vi "UHR-Fleezers Control (host) - 10.2.vi"() -> ()   [LabVIEW 2009] (continued)
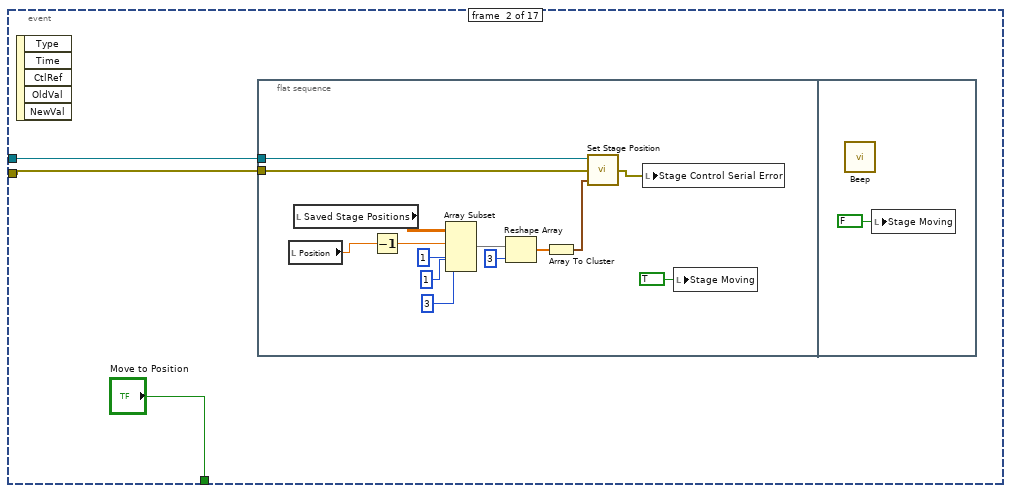
[diagram p2: hidden frame]
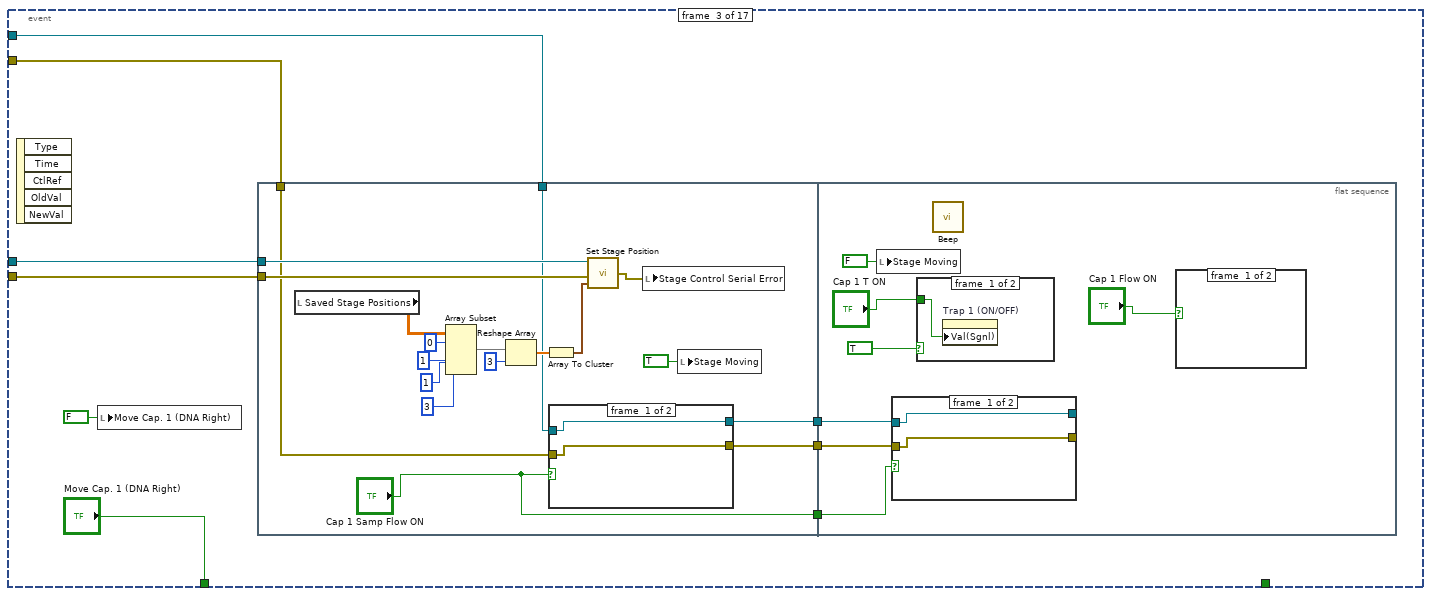
[diagram p3: hidden frame]
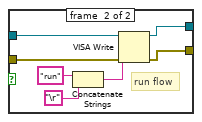
[diagram p4: hidden frame]
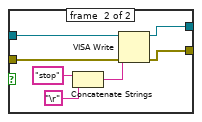
[diagram p5: hidden frame]
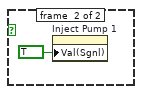
[diagram p6: hidden frame]
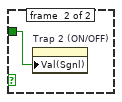
[diagram p7: hidden frame]
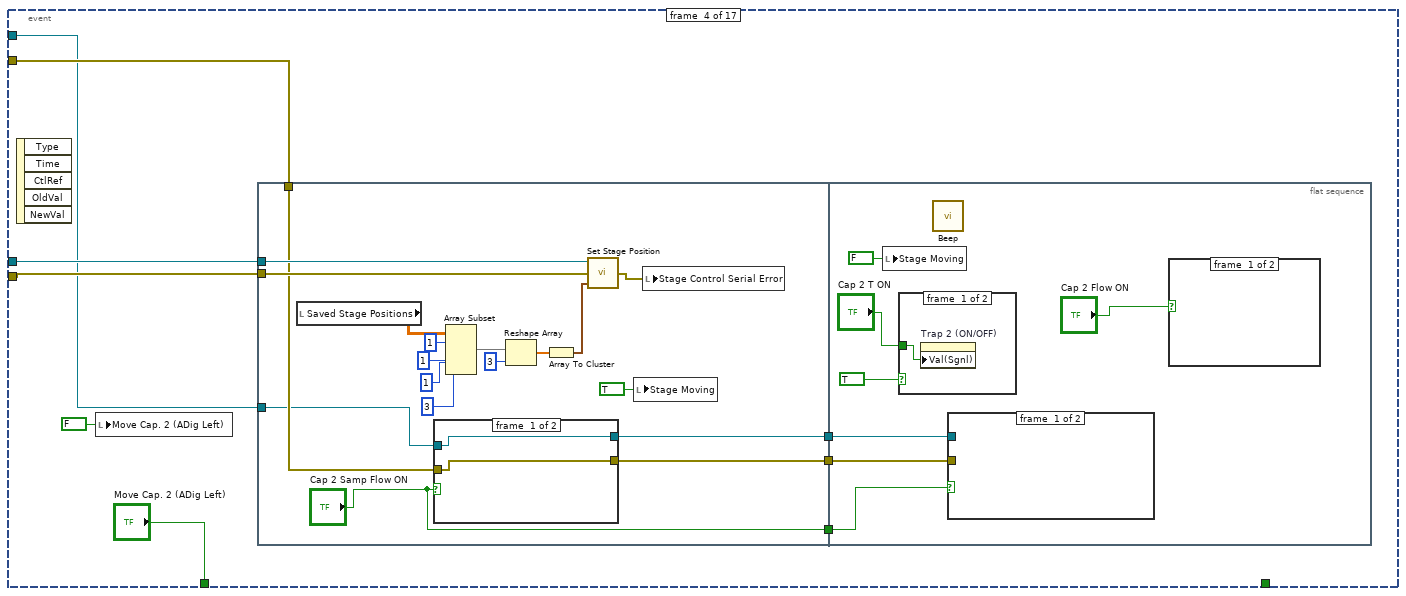
[diagram p8: hidden frame]
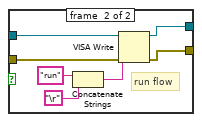
[diagram p9: hidden frame]
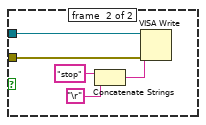
[diagram p10: hidden frame]
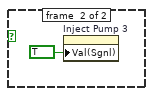
[diagram p11: hidden frame]
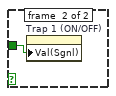
[diagram p12: hidden frame]
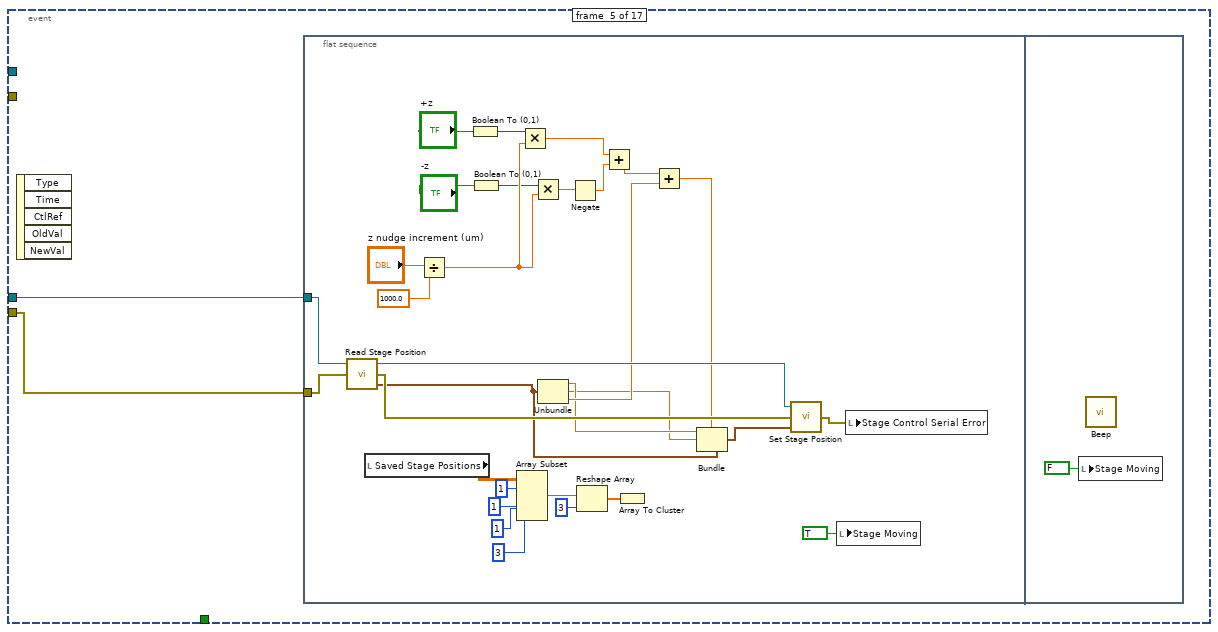
[diagram p13: hidden frame]
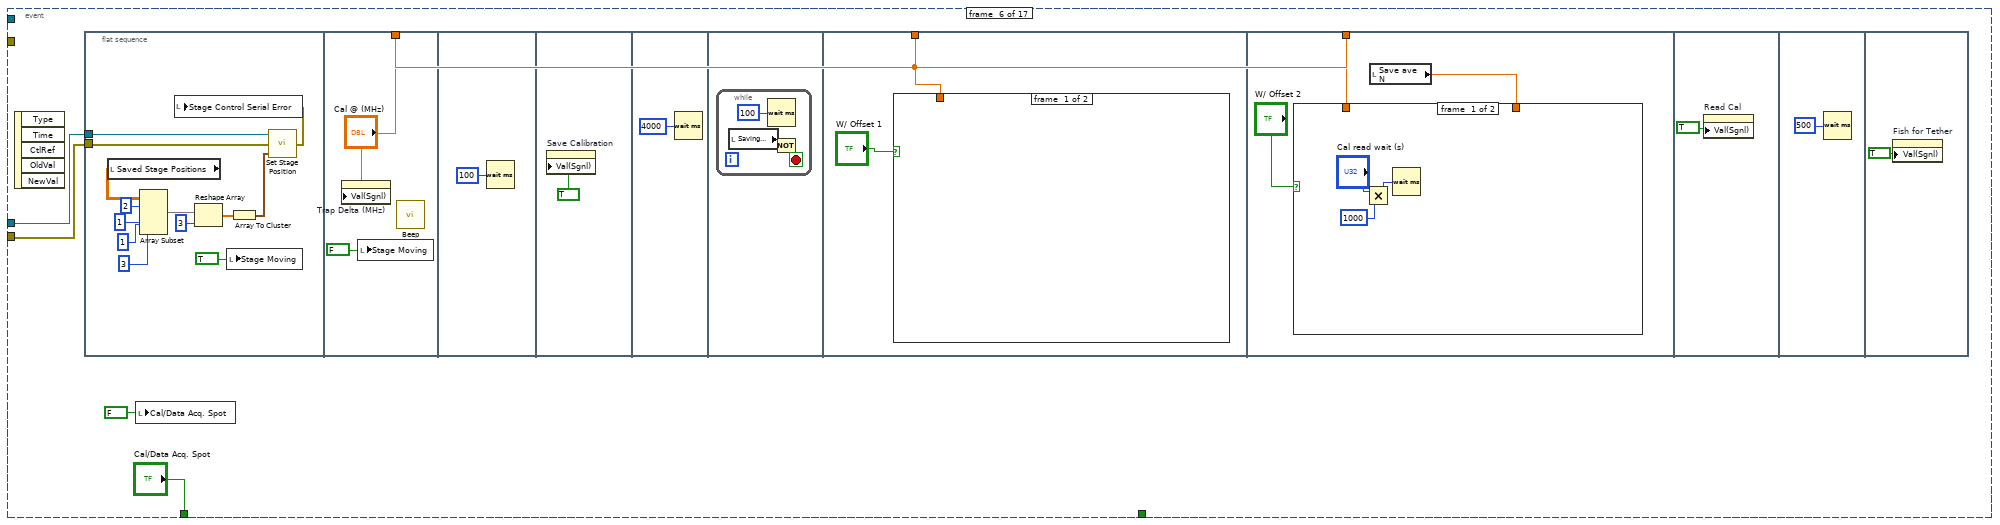
[diagram p14: hidden frame]
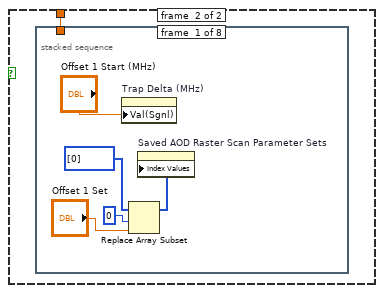
[diagram p15: hidden frame]
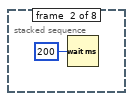
[diagram p16: hidden frame]
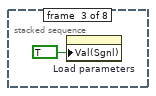
[diagram p17: hidden frame]
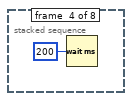
[diagram p18: hidden frame]
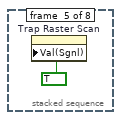
[diagram p19: hidden frame]
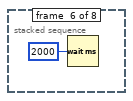
[diagram p20: hidden frame]
              frame #0 {
              }
              frame #1 {
                n2014 = call "IMAQ AVI Close"("Avi Refnum"=w8057) -> ()  [unwired: 1 in, 10 out]
              }
            }
            n2015 = call "IMAQ AVI Create"("Frames Per Second"=u32 30, "AVI Path"=w8046) -> ("Avi Refnum"=w8054:T48)  [unwired: 5 in, 4 out]
            n2016 = local write "Video Index"(w8056) -> ()
          }
        }
        n2017 = Equal To 0?(x=w8037) -> (x = 0?=w8036:bool)
        n2018 = Select(t=w8027, s=w8028, f=w8025) -> (s? t:f=w8026:T48)
        n2019 = case shown="True" w8036 {
          tunnel: w8035 -> [w8058 w8083]
          tunnel: w8034 -> [_ w8082]
          tunnel: [w8058 w8079] -> w8032
          tunnel: w8031 -> [_ w8063]
          tunnel: w8020 -> [_ w8067]
          tunnel: w8026 -> [_ w8065]
          tunnel: w8018 -> [_ w8060]
          tunnel: w8017 -> [_ w8059]
          frame #0 {
          }
          frame #1 {
            w8073 = u32 0 ("X-offset IN")
            n2020 = call "DMR_GetImageRequestBufferData.vi"("driver handle IN"=w8083, "request number IN"=w8082) -> ("width OUT"=w8072:i32, "height OUT"=w8071:i32, "driver handle OUT"=w8078:i32, "request number OUT"=w8077:i32, "bytes per pixel OUT"=w8074:i32)  [unwired: 13 out]
            n2021 = call "DMR_GetImageRequestBufferImageData.vi"("driver handle IN"=w8078, "request number IN"=w8077, "bytes per pixel IN"=w8074, "X-offset IN"=w8073, "Y-offset IN"=w8073, "height IN"=w8071, "width IN"=w8072) -> ("driver handle OUT"=w8076:u32, "request number OUT"=w8075:u32, "image OUT"=w8068:u32[][])  [unwired: 10 out]
            n2022 = call "DMR_ImageRequestUnlock.vi"("request number IN"=w8075, "driver handle IN"=w8076) -> ("driver handle OUT"=w8081:i32)  [unwired: 1 in, 2 out]
            n2023 = case shown="True" "Averaging" {
              tunnel: w8068 -> [w8119 w8124]
              tunnel: [w8119 w8123] -> w8064
              tunnel: w8067 -> [_ w8121]
              frame #0 {
              }
              frame #1 {
                (unwired) 1
                w8129 = 1
                n2024 = feedback #32(w8121) -> (w8120:u32[][])
                n2025 = Add(x=w8124, y=w8120) -> (x+y=w8125:u32[][])
                n2026 = Select(t=w8121, s="Reset Averaging", f=w8125) -> (s? t:f=w8127:u32[][])
                n2027 = feedback #33(w8129) -> (w8122:i32)
                n2028 = Divide(x=w8125, y=w8122) -> (x/y=w8126:dbl[][])
                n2029 = Increment(x=w8122) -> (x+1=w8130:i32)
                n2030 = To Unsigned Long Integer(number=w8126) -> (unsigned 32bit integer=w8123:u32[][])
                n2031 = Select(t=w8129, s="Reset Averaging", f=w8130) -> (s? t:f=w8128:i32)
              }
            }
            n2032 = call "DMR_ImageRequestSingle.vi"("request control IN"=0, "driver handle IN"=w8081) -> ("driver handle OUT"=w8079:i32)  [unwired: 3 out]
            n2033 = disable-structure shown="Disabled" {
              disable-tunnel: w8064 -> [w8096 _]
              disable-tunnel: w8060 -> [w8095 _]
              frame #0 {
                n2034 = To Double Precision Float(number=w8096) -> (double precision float=w8094:dbl[][])
                n2035 = In Range and Coerce(upper limit="Intensity Upper", x=w8094, lower limit="Intensity Lower") -> (coerced(x)=w8093:dbl[][])  [unwired: 1 out]
                n2036 = Subtract(x="Intensity Upper", y="Intensity Lower") -> (x-y=w8090:dbl)
                n2037 = Subtract(x=w8093, y="Intensity Lower") -> (x-y=w8091:dbl[][])
                n2038 = Divide(x=w8091, y=w8090) -> (x/y=w8092:dbl[][])
                n2039 = Multiply(x=255.0, y=w8092) -> (x*y=w8088:dbl[][])
                n2040 = To Unsigned Byte Integer(number=w8088) -> (unsigned 8bit integer=w8097:u8[][])
                n2041 = call "IMAQ ArrayToImage"("Image Pixels (U8)"=w8097, "Image"=w8095) -> ("Image Out"=w8084:T2)  [unwired: 4 in, 5 out]
                n2042 = First Call?() -> (First Call?: T/F=w8085:bool)
                n2043 = case shown="True" w8085 {
                  tunnel: w8084 -> [w8098 w8109]
                  frame #0 {
                    n2044 = flat-sequence {
                      tunnel: w8098 -> [w8104]
                      frame #0 {
                        w8101 = FALSE ("Get/Set Status? (Set)")
                        w8100 = 0 ("Window Number (0...15)")
                        n2045 = call "IMAQ WindSize"("Get/Set Status? (Set)"=w8101, "Window Number"=w8100) -> ("Width & Height out"=→"Window Size":cluster{"Width":i32, "Height":i32})  [unwired: 4 in, 2 out]
                        n2046 = call "IMAQ WindMove"("Window Number (0...15)"=w8100, "Get/Set Status? (Set)"=w8101) -> ("Coordinates (screen)"=→"Window Position":cluster{"X Position":i32, "Y Position":i32})  [unwired: 3 in, 1 out]
                        n2047 = call "IMAQ WindDraw"("Resize to Image Size? (Y)"=FALSE, "Window Number (0...15)"=w8100, "Image"=w8104) -> ()  [unwired: 7 in, 2 out]
                      }
                      frame #1 {
                        n2048 = call "IMAQ WindZoom 2"("Center Point"="Center Point", "Zoom to Fit? (False)"=FALSE, "Zoom Factor"="Zoom Factor") -> ()  [unwired: 5 in, 4 out]
                      }
                    }
                  }
                  frame #1 {
                    n2049 = flat-sequence {
                      tunnel: w8109 -> [w8112]
                      tunnel: [w8110] -> w8108
                      tunnel: w8108 -> [w8114]
                      frame #0 {
                        w8111 = TRUE ("Resize to Image Size? (Y)")
                        w8110 = 0 ("Window Number (0...15)")
                        n2050 = call "IMAQ WindNonTearing"("Window Number"=w8110, "NonTearing? (True)"=w8111) -> ()  [unwired: 8 in, 2 out]
                        n2051 = call "IMAQ WindDraw"("Resize to Image Size? (Y)"=w8111, "Window Number (0...15)"=w8110, "Image"=w8112) -> ()  [unwired: 7 in, 2 out]
                      }
                      frame #1 {
                        n2052 = call "IMAQ WindSize"("Scrollbars? (N)"=FALSE, "Width & Height"="Initial Window Size", "Window Number"=w8114) -> ()  [unwired: 3 in, 3 out]
                        n2053 = call "IMAQ WindMove"("Window Number (0...15)"=w8114, "Coordinates (screen)"="Initial Window Position") -> ()  [unwired: 3 in, 2 out]
                      }
                    }
                  }
                }
              }
              frame #1 {
              }
            }
            n2054 = To Unsigned Byte Integer(number=w8064) -> (unsigned 8bit integer=w8062:u8[][])
            n2055 = call "IMAQ ArrayToImage"("Image Pixels (U8)"=w8062, "Image"=w8063) -> ("Image Out"=w8061:T2)  [unwired: 4 in, 5 out]
            "Primary Video Display" <- w8061
            n2056 = case shown="True" "Save Video" {
              tunnel: w8065 -> [_ w8118]
              tunnel: w8061 -> [_ w8117]
              frame #0 {
              }
              frame #1 {
                n2057 = call "IMAQ AVI Write Frame"("Image"=w8117, "Avi Refnum"=w8118) -> ()  [unwired: 2 in, 8 out]
              }
            }
            n2058 = case shown="True" "Save Image" {
              tunnel: w8062 -> [_ w8133]
              tunnel: w8059 -> [_ w8132]
              frame #0 {
              }
              frame #1 {
                n2059 = call <vilib>:"Flatten Pixmap.vi"("colors"=w8132, "8-bit pixmap"=w8133) -> ("image data"=w8139:T49)  [unwired: 4 in, 5 out]
                n2060 = call "Create new save file.vi"("Insert"="video_frame_" ("string"), "Ext"=".bmp" ("string"), "Index In"="Image Index") -> ("Path Out"=w8135:path, "Index Out"=w8140:dbl)
                n2061 = Increment(x=w8140) -> (x+1=w8134:dbl)
                n2062 = local write "Image Index"(w8134) -> ()
                n2063 = call <vilib>:"Write BMP File.vi"("image data"=w8139, "path to BMP file"=w8135) -> ()  [unwired: 1 in, 9 out]
              }
            }
          }
        }
        n2064 = node-c288(w8021) -> ()  [unwired: 1 out]
      }
      n2065 = node-c288(w8005) -> ()  [unwired: 1 out]
      n2066 = call "DMR_CloseDevice.vi"("driver handle IN"=w8010) -> ()  [unwired: 1 in, 4 out]
    }
    frame #4 {
      n2067 = call "DMR_Close.vi"() -> ()  [unwired: 1 out]
    }
  }
  n2068 = timed-loop "Oscillate AOD (debugging)" {
    tunnel: w8 -> [w8146]
    tunnel: [w8145] -> w53
    timing: w48 -> [_]
    timing-out: [_] -> w47
    stop <- w8145 stop-if-true
    n2069 = node-c288() -> ()  [unwired: 2 out]
    n2070 = event shown="[0] \"Oscillate Set 1\", \"Fish for Tether\": Value Change" {
      selector: _ -> [_ _ _]
      dyn-events: _ -> [_ _ _]
      timeout: _ -> [_ _ _]
      tunnel: w8146 -> [w8153 _ _]
      tunnel: [FALSE ("Stop All") _ w8421] -> w8145
      event #0 {
        n2071 = event-data() -> ()  [unwired: 6 out]
        n2072 = local read "Oscillate Set 1"() -> (w8152:bool)
        n2073 = Or(x=w8152, y="Fish for Tether") -> (x .or. y?=w8150:bool)
        n2074 = case shown="True" w8150 {
          tunnel: w8153 -> [_ w8155]
          tunnel: "Fish for Tether" -> [_ w8154]
          frame #0 {
          }
          frame #1 {
            n2075 = case shown="True" w8154 {
              frame #0 {
              }
              frame #1 {
                n2076 = local write "Scan axis 2"(TRUE) -> ()
                n2077 = local write "Tether"(FALSE ("Tether")) -> ()
              }
            }
            n2078 = node-c288() -> (w8157:T23)  [unwired: 4 out]
            n2079 = timed-loop "Oscillate AOD" {
              timing: w8157 -> [_]
              timing-out: [_] -> w8156
              tunnel: w8155 -> [w8167]
              tunnel: w8154 -> [w8166]
              i -> [w8169]
              stop <- w8165 stop-if-true
              n2080 = node-c288() -> (w8168:i64)  [unwired: 1 out]
              n2081 = flat-sequence {
                tunnel: w8169 -> [w8196]
                tunnel: w8168 -> [w8195]
                tunnel: w8167 -> [w8174]
                tunnel: w8166 -> [w8177]
                tunnel: [w8177] -> w8164
                tunnel: [w8176] -> w8163
                tunnel: [w8173] -> w8162
                tunnel: [w8170] -> w8160
                tunnel: w8164 -> [w8232]
                tunnel: w8163 -> [w8230]
                tunnel: w8162 -> [w8229]
                tunnel: [w8228] -> w8161
                tunnel: w8160 -> [w8227]
                tunnel: [w8295] -> w8165
                tunnel: w8161 -> [w8294]
                frame #0 {
                  n2082 = Divide(x=w8195, y=i64 1000) -> (x/y=w8190:dbl)
                  n2083 = Multiply(x=w8190, y=w8196) -> (x*y=w8192:dbl)
                  n2084 = local read "BD 1 Frequency 2 (MHz)"() -> (w8175:dbl)
                  n2085 = Multiply(x="Osc. freq. (Hz)", y=6.283185307179586) -> (x*y=w8193:dbl)
                  n2086 = Multiply(x=w8193, y=w8192) -> (x*y=w8172:dbl)
                  n2087 = local read "BD 1 Frequency 1 (MHz)"() -> (w8180:dbl)
                  n2088 = case shown="True" w8177 {
                    tunnel: w8172 -> [w8202 w8207]
                    tunnel: w8180 -> [_ w8218]
                    tunnel: w8175 -> [_ w8219]
                    tunnel: [w8199 w8213] -> w8178
                    tunnel: [FALSE w8210] -> w8173
                    tunnel: [0.0 w8203] -> w8170
                    frame #0 {
                      n2089 = Sine(x=w8202) -> (sin(x)=w8200:dbl)
                      n2090 = Multiply(x=w8200, y="Osc. amp. (MHz)") -> (x*y=w8199:dbl)
                    }
                    frame #1 {
                      n2091 = Cosine(x=w8207) -> (cos(x)=w8222:dbl)
                      n2092 = Subtract(x=w8219, y=w8218) -> (x-y=w8217:dbl)
                      n2093 = Decrement(x=w8222) -> (x-1=w8221:dbl)
                      n2094 = Subtract(x=w8217, y="Closest Delta (MHz)") -> (x-y=w8214:dbl)
                      n2095 = Divide(x=w8221, y=-2.0) -> (x/y=w8215:dbl)
                      n2096 = Multiply(x=w8215, y=w8214) -> (x*y=w8213:dbl)
                      n2097 = local read "Vec Mean of T1 T2"() -> (w8209:dbl[])
                      n2098 = Greater?(x=w8209, y="Stop F (pN)") -> (0:w8211:bool[])
                      n2099 = Or Array Elements(Boolean array=w8211) -> (logical OR=w8210:bool)
                      n2100 = Divide(x=w8207, y=6.283185307179586) -> (x/y=w8206:dbl)
                      n2101 = Round Toward +Infinity(x=w8206) -> (ceil(x): smallest int >= x=w8203:dbl)
                      "Attempts" <- w8203
                      n2102 = Greater?(x=w8203, y="Attempt Limit") -> (0:w8205:bool)
                      n2103 = case shown="True" w8205 {
                        frame #0 {
                        }
                        frame #1 {
                          n2104 = call <vilib>:"Beep.vi"() -> ()  [unwired: 3 in, 9 out]
                          n2105 = local write "Fish for Tether"(FALSE ("Fish for Tether")) -> ()
                          n2106 = local read "Messages"() -> (w8224:string)
                          n2107 = call "Update messages.vi"("Message to add"="Tether fishing timeout." ("Messages"), "Old message string"=w8224) -> ("New message string"=→"Messages":string)
                        }
                      }
                    }
                  }
                  n2108 = local read "BD 2 Frequency 1 (MHz)"() -> (w8179:dbl)
                  n2109 = Select(t=w8180, s="Scan axis 2", f=w8179) -> (s? t:f=w8183:dbl)
                  n2110 = Add(x=w8178, y=w8183) -> (x+y=w8176:dbl)
                  n2111 = Select(t=w8176, s="Scan axis 2", f=w8180) -> (s? t:f=w8186:dbl)
                  n2112 = Select(t=w8179, s="Scan axis 2", f=w8176) -> (s? t:f=w8185:dbl)
                  n2113 = local read "Y RF Frequency Limits (MHz)"() -> (w8181:T16)
                  n2114 = local read "X RF Frequency Limits (MHz)"() -> (w8182:T16)
                  n2115 = local read "BD 1 Frequency 3 (MHz)"() -> (w8189:dbl)
                  n2116 = local read "BD 2 Frequency 2 (MHz)"() -> (w8188:dbl)
                  n2117 = local read "BD 2 Frequency 3 (MHz)"() -> (w8187:dbl)
                  n2118 = call "set RF board frequency - interlace.vi"("Board 2 Frequency Limits"=w8181, "Board 1 Frequency Limits"=w8182, "FPGA VI Reference In"=w8174, "Board 2 Frequency 3 (MHz)"=w8187, "Board 1 Frequency 3 (MHz)"=w8189, "Board 2 Frequency 2 (MHz)"=w8188, "Board 2 Frequency 1 (MHz)"=w8185, "Board 1 Frequency 2 (MHz)"=w8175, "Board 1 Frequency 1  (MHz)"=w8186) -> ()  [unwired: 1 in, 2 out]
                }
                frame #1 {
                  n2119 = And(x=w8232, y=w8229) -> (x .and. y?=w8231:bool)
                  n2120 = case "Only if were fishing and now formed tether" shown="True" w8231 {
                    tunnel: w8230 -> [w8234 w8247]
                    tunnel: [w8233 w8246] -> w8228
                    tunnel: w8227 -> [_ w8242]
                    frame #0 {
                      n2121 = local read "Fish for Tether"() -> (w8233:bool)
                      n2122 = case shown="False" w8233 {
                        tunnel: w8234 -> [w8235 _]
                        frame #0 {
                          n2123 = property on="BD 1 Frequency 1 (MHz)" class="DigNum (strict)"("Val(Sgnl)"=w8235) -> ()  [unwired: 2 in, 2 out]
                        }
                        frame #1 {
                        }
                      }
                    }
                    frame #1 {
                      w8246 = FALSE ("Fish for Tether")
                      n2124 = call <vilib>:"Beep.vi"() -> ()  [unwired: 3 in, 9 out]
                      n2125 = Number To Decimal String(number=w8242, width (-)=i16 1) -> (decimal integer string=w8240:string)
                      n2126 = case shown="\"2\", \"3\", \"4\", \"5\", \"6\"" "Then..." {
                        selector: "Then..." -> [_ w8250]
                        tunnel: w8247 -> [w8249 _]
                        frame #0 {
                          n2127 = property on="BD 1 Frequency 1 (MHz)" class="DigNum (strict)"("Val(Sgnl)"=w8249) -> ()  [unwired: 2 in, 2 out]
                        }
                        frame #1 {
                          n2128 = flat-sequence {
                            tunnel: w8250 -> [w8252]
                            frame #0 {
                              n2129 = property on="Trap Delta (MHz)" class="DigNum (strict)"("Val(Sgnl)"="Move to Delta 1 (MHz)") -> ()  [unwired: 2 in, 2 out]
                            }
                            frame #1 {
                              n2130 = case shown="\"5\", \"6\"" w8252 {
                                selector: w8252 -> [w8255 w8265 _]
                                frame #0 {
                                n2131 = flat-sequence {
                                tunnel: w8255 -> [w8256]
                                tunnel: [w8256] -> w8253
                                tunnel: [w8258] -> w8254
                                tunnel: w8253 -> [w8258]
                                tunnel: w8254 -> [w8262]
                                frame #0 {
                                n2132 = property on="Green Laser ON/Interlacing" class="Bool (strict)"("Val(Sgnl)"=TRUE ("Value (Signaling)")) -> ()  [unwired: 2 in, 2 out]
                                }
                                frame #1 {
                                n2133 = Multiply(x="Wait Before Save (s)", y=u32 1000 ("x")) -> (x*y=w8260:u32)
                                n2134 = Wait (ms)(milliseconds to wait=w8260) -> ()  [unwired: 1 out]
                                }
                                frame #2 {
                                n2135 = property on="Start Saving" class="Bool (strict)"("Value"=TRUE ("Start Saving")) -> ()  [unwired: 2 in, 2 out]
                                n2136 = case shown="\"4\"" w8262 {
                                frame #0 {
                                }
                                frame #1 {
                                n2137 = property on="Fl. Triggered..." class="Bool (strict)"("Val(Sgnl)"=TRUE ("Value (Signaling)")) -> ()  [unwired: 2 in, 2 out]
                                }
                                }
                                }
                                }
                                }
                                frame #1 {
                                n2138 = stacked-sequence {
                                tunnel: w8265 -> [_ _ _ _ _ _ _ _ w8282 _ _]
                                frame #0 {
                                n2139 = Replace Array Subset(array=u32[] [0] ("Index Values"), new element="Raster Set Upon Tether", index=0) -> (w8266:u32[])
                                n2140 = property on="Saved AOD Raster Scan Parameter Sets" class="Arr (strict)"("Index Values"=w8266) -> ()  [unwired: 2 in, 2 out]
                                }
                                frame #1 {
                                n2141 = Wait (ms)(milliseconds to wait=u32 500) -> ()  [unwired: 1 out]
                                }
                                frame #2 {
                                n2142 = property on="Load parameters" class="Bool (strict)"("Val(Sgnl)"=TRUE ("Value (Signaling)")) -> ()  [unwired: 2 in, 2 out]
                                }
                                frame #3 {
                                n2143 = Wait (ms)(milliseconds to wait=u32 500) -> ()  [unwired: 1 out]
                                }
                                frame #4 {
                                n2144 = property on="Trap Raster Scan" class="Bool (strict)"("Val(Sgnl)"=TRUE ("Value (Signaling)")) -> ()  [unwired: 2 in, 2 out]
                                }
                                frame #5 {
                                n2145 = Wait (ms)(milliseconds to wait=u32 2000) -> ()  [unwired: 1 out]
                                }
                                frame #6 {
                                n2146 = while {
                                stop <- w8277 stop-if-true
                                n2147 = local read "Raster Scanning..."() -> (w8276:bool)
                                n2148 = local read "Saving..."() -> (w8279:bool)
                                n2149 = Wait (ms)(milliseconds to wait=u32 100) -> ()  [unwired: 1 out]
                                n2150 = Not(x=w8279) -> (.not. x?=w8278:bool)
                                n2151 = Not(x=w8276) -> (.not. x?=w8275:bool)
                                n2152 = And(x=w8278, y=w8275) -> (x .and. y?=w8277:bool)
                                }
                                }
                                frame #7 {
                                n2153 = property on="Trap Delta (MHz)" class="DigNum (strict)"("Val(Sgnl)"="Move to Delta 2 (MHz)") -> ()  [unwired: 2 in, 2 out]
                                }
                                frame #8 {
                                n2154 = local read "Tether"() -> (w8283:bool)
                                n2155 = case shown="True" w8283 {
                                tunnel: w8282 -> [_ w8284]
                                frame #0 {
                                }
                                frame #1 {
                                n2156 = flat-sequence {
                                tunnel: w8284 -> [w8286]
                                frame #0 {
                                n2157 = Wait (ms)(milliseconds to wait=u32 500) -> ()  [unwired: 1 out]
                                }
                                frame #1 {
                                n2158 = case shown="\"6\"" w8286 {
                                frame #0 {
                                }
                                frame #1 {
                                n2159 = property on="Green Laser ON/Interlacing" class="Bool (strict)"("Val(Sgnl)"=TRUE ("Green Laser ON/Interlacing")) -> ()  [unwired: 2 in, 2 out]
                                }
                                }
                                }
                                frame #2 {
                                n2160 = Wait (ms)(milliseconds to wait=u32 500) -> ()  [unwired: 1 out]
                                }
                                frame #3 {
                                n2161 = local write "Start Saving"("Save at end (5, 6)") -> ()
                                }
                                }
                                }
                                }
                                }
                                frame #9 {
                                n2162 = local read "Bead Sep. Int. Time (s)"() -> (w8292:dbl)
                                n2163 = Multiply(x=w8292, y=1000.0) -> (x*y=w8291:dbl)
                                n2164 = Wait (ms)(milliseconds to wait=w8291) -> ()  [unwired: 1 out]
                                }
                                frame #10 {
                                n2165 = property on="Rescale on Mean" class="Bool (strict)"("Val(Sgnl)"=TRUE ("Value (Signaling)")) -> ()  [unwired: 2 in, 2 out]
                                }
                                }
                                }
                                frame #2 {
                                }
                              }
                            }
                          }
                        }
                      }
                      n2166 = Concatenate Strings("Formed tether in ", w8240, " attempt(s)." ("string")) -> (w8237:string)
                      n2167 = local read "Messages"() -> (w8244:string)
                      n2168 = local write "Fish for Tether"(w8246) -> ()
                      n2169 = call "Update messages.vi"("Message to add"=w8237, "Old message string"=w8244) -> ("New message string"=w8243:string)
                      n2170 = local write "Messages"(w8243) -> ()
                      n2171 = Get Date/Time In Seconds() -> (seconds since 1Jan1904=→"Time tether formed":timestamp)
                      "Tether" <- "Tether Alarm?"
                    }
                  }
                }
                frame #2 {
                  n2172 = local read "Oscillate Set 1"() -> (w8299:bool)
                  n2173 = Or(x=w8299, y=w8294) -> (x .or. y?=w8296:bool)
                  n2174 = local read "Stop All"() -> (w8297:bool)
                  n2175 = Not(x=w8296) -> (.not. x?=w8298:bool)
                  n2176 = Compound Arithmetic op=OR(w8297, w8298) -> (w8295:bool)
                }
              }
              n2177 = node-c288() -> ()  [unwired: 2 out]
            }
            n2178 = node-c288(w8156) -> ()  [unwired: 1 out]
          }
        }
      }
      event #1 {
        n2179 = event-data() -> ()  [unwired: 7 out]
        n2180 = case shown="True" "Fl. Triggered..." {
          frame #0 {
          }
          frame #1 {
            n2181 = node-c288() -> (w8309:T23)  [unwired: 4 out]
            n2182 = timed-loop {
              timing: w8309 -> [_]
              timing-out: [_] -> w8308
              tunnel: "Action" -> [w8313]
              shift-right: [w8310] -> _
              shift-left: u8 255 -> [w8312]
              stop <- w8314 stop-if-true
              n2183 = node-c288() -> ()  [unwired: 2 out]
              n2184 = flat-sequence {
                tunnel: w8313 -> [w8326]
                tunnel: w8312 -> [w8323]
                tunnel: [w8322] -> w8311
                tunnel: [w8412] -> w8314
                tunnel: w8311 -> [w8411]
                tunnel: [w8411] -> w8310
                frame #0 {
                  n2185 = local read "Delta Fl. 2"() -> (w8317:dbl)
                  n2186 = local read "Delta Fl. 1"() -> (w8318:dbl)
                  n2187 = Select(t=w8318, s="APD to Watch", f=w8317) -> (s? t:f=w8316:dbl)
                  n2188 = Multiply(x="Fl. Delta Thresh. (kHz)", y=1000.0) -> (x*y=w8325:dbl)
                  n2189 = Greater?(x=w8316, y=w8325) -> (0:w8320:bool)
                  n2190 = Or(x="Force Yank", y=w8320) -> (x .or. y?=w8321:bool)
                  n2191 = case shown="True" w8321 {
                    tunnel: w8326 -> [_ w8336]
                    tunnel: w8323 -> [w8328 w8332]
                    tunnel: [w8328 w8329] -> w8322
                    frame #0 {
                    }
                    frame #1 {
                      n2192 = flat-sequence {
                        tunnel: w8333 -> [w8342]
                        tunnel: [w8342] -> w8337
                        tunnel: w8336 -> [w8341]
                        tunnel: [w8341] -> w8335
                        tunnel: [w8340] -> w8334
                        tunnel: w8332 -> [w8339]
                        tunnel: [w8338] -> w8331
                        tunnel: w8337 -> [w8367]
                        tunnel: w8335 -> [w8366]
                        tunnel: w8334 -> [w8365]
                        tunnel: w8331 -> [w8364]
                        tunnel: [w8364] -> w8330
                        tunnel: w8330 -> [w8409]
                        tunnel: [w8409] -> w8329
                        frame #0 {
                          n2193 = call <vilib>:"Beep.vi"() -> ()  [unwired: 3 in, 9 out]
                          n2194 = local write "Waiting"(FALSE ("Waiting")) -> ()
                          n2195 = Increment(x=w8339) -> (x+1=w8338:u8)
                          n2196 = case shown="\"Yank\"" w8341 {
                            tunnel: w8338 -> [_ _ w8348]
                            frame #0 {
                              n2197 = property on="Confocal Image" class="Bool (strict)"("Val(Sgnl)"=TRUE ("Value (Signaling)")) -> ()  [unwired: 2 in, 2 out]
                            }
                            frame #1 {
                            }
                            frame #2 {
                              n2198 = flat-sequence {
                                tunnel: w8348 -> [w8351]
                                tunnel: [w8350] -> w8347
                                tunnel: ["N Array El"] -> w8346
                                tunnel: w8347 -> [w8361]
                                tunnel: w8346 -> [w8357]
                                frame #0 {
                                n2199 = Multiply(x="Yank Delay (s)", y=1000.0) -> (x*y=w8354:dbl)
                                n2200 = Quotient & Remainder(x=w8351, y="N Array El") -> (x-y*floor(x/y)=w8350:u8)  [unwired: 1 out]
                                n2201 = Wait (ms)(milliseconds to wait=w8354) -> ()  [unwired: 1 out]
                                }
                                frame #1 {
                                n2202 = Random Number (0-1)() -> (number: 0 to 1=w8358:dbl)
                                n2203 = Multiply(x=w8357, y=w8358) -> (x*y=w8356:dbl)
                                n2204 = Round Toward -Infinity(1:w8356) -> (0:w8355:dbl)
                                n2205 = Select(t=w8355, s="Random Choice", f=w8361) -> (s? t:f=w8359:dbl)
                                n2206 = Index Array(array="Yank to Delta Array (MHz)", index=w8359) -> (element=w8362:dbl)
                                n2207 = property on="Trap Delta (MHz)" class="DigNum (strict)"("Val(Sgnl)"=w8362) -> ()  [unwired: 2 in, 2 out]
                                }
                              }
                            }
                          }
                          n2208 = local read "Time (s)"() -> (w8340:dbl)
                          "Fl. High" <- TRUE ("Yanking")
                        }
                        frame #1 {
                          n2209 = node-c288() -> (w8369:T23)  [unwired: 4 out]
                          n2210 = timed-loop {
                            timing: w8369 -> [_]
                            timing-out: [_] -> w8368
                            tunnel: w8367 -> [w8385]
                            tunnel: w8366 -> [w8383]
                            tunnel: w8365 -> [w8382]
                            stop <- w8384 stop-if-true
                            n2211 = node-c288() -> ()  [unwired: 2 out]
                            n2212 = local read "Fl. Delta Thresh. (kHz)"() -> (w8377:dbl)
                            n2213 = local read "Fl. Triggered..."() -> (w8386:bool)
                            n2214 = local read "Delta Fl. 1"() -> (w8373:dbl)
                            n2215 = local read "Delta Fl. 2"() -> (w8371:dbl)
                            n2216 = local read "Stop All"() -> (w8380:bool)
                            n2217 = local read "APD to Watch"() -> (w8372:bool)
                            n2218 = Select(t=w8373, s=w8372, f=w8371) -> (s? t:f=w8370:dbl)
                            n2219 = Not(x=w8386) -> (.not. x?=w8381:bool)
                            n2220 = Multiply(x=w8377, y=1000.0) -> (x*y=w8376:dbl)
                            n2221 = Negate(x=w8376) -> (-x=w8375:dbl)
                            n2222 = Less?(x=w8370, y=w8375) -> (x < y?=w8379:bool)
                            n2223 = Compound Arithmetic op=OR(w8379, w8380, w8381, "Force Reset") -> (w8384:bool)
                            n2224 = case shown="True" w8384 {
                              tunnel: w8385 -> [_ w8397]
                              tunnel: w8383 -> [_ w8396]
                              tunnel: w8382 -> [_ w8394]
                              frame #0 {
                              }
                              frame #1 {
                                n2225 = case shown="\"Yank\"" w8396 {
                                tunnel: w8397 -> [_ w8398]
                                frame #0 {
                                }
                                frame #1 {
                                n2226 = flat-sequence {
                                tunnel: [w8403] -> w8399
                                tunnel: w8398 -> [w8403]
                                tunnel: w8399 -> [w8404]
                                frame #0 {
                                n2227 = local read "Yank Delay (s)"() -> (w8402:dbl)
                                n2228 = Multiply(x=w8402, y=1000.0) -> (x*y=w8400:dbl)
                                n2229 = Wait (ms)(milliseconds to wait=w8400) -> ()  [unwired: 1 out]
                                }
                                frame #1 {
                                n2230 = property on="Trap Delta (MHz)" class="DigNum (strict)"("Val(Sgnl)"=w8404) -> ()  [unwired: 2 in, 2 out]
                                }
                                }
                                }
                                }
                                n2231 = local read "Time (s)"() -> (w8395:dbl)
                                n2232 = Subtract(x=w8395, y=w8394) -> (x-y=w8391:dbl)
                                "Duration (s)" <- w8391
                                n2233 = Number To Decimal String(number=w8391, width (-)=i16 0) -> (decimal integer string=w8389:string)
                                n2234 = Concatenate Strings(w8389, " s fluorescence event." ("string")) -> (w8387:string)
                                n2235 = local read "Messages"() -> (w8393:string)
                                n2236 = call "Update messages.vi"("Message to add"=w8387, "Old message string"=w8393) -> ("New message string"=w8392:string)
                                n2237 = call <vilib>:"Beep.vi"() -> ()  [unwired: 3 in, 9 out]
                                n2238 = local write "Messages"(w8392) -> ()
                              }
                            }
                            n2239 = node-c288() -> ()  [unwired: 2 out]
                          }
                          n2240 = node-c288(w8368) -> ()  [unwired: 1 out]
                        }
                        frame #2 {
                          n2241 = local write "Fl. High"(FALSE ("Yanking")) -> ()
                        }
                      }
                      n2242 = local read "Trap Delta (MHz)"() -> (w8333:dbl)
                    }
                  }
                }
                frame #1 {
                  n2243 = local read "Stop All"() -> (w8415:bool)
                  n2244 = local read "Fl. Triggered..."() -> (w8413:bool)
                  n2245 = Not(x=w8413) -> (.not. x?=w8414:bool)
                  n2246 = Or(x=w8414, y=w8415) -> (x .or. y?=w8412:bool)
                  n2247 = Not(x=w8412) -> (.not. x?=→"Waiting":bool)
                }
              }
              n2248 = node-c288() -> ()  [unwired: 2 out]
            }
            n2249 = node-c288(w8308) -> ()  [unwired: 1 out]
          }
        }
      }
      event #2 {
        n2250 = event-data() -> ()  [unwired: 7 out]
        n2251 = local read "Stop All"() -> (w8421:bool)
      }
    }
    n2252 = node-c288() -> ()  [unwired: 2 out]
  }
  n2253 = node-c288(w49) -> ()  [unwired: 1 out]
  n2254 = node-c288(w36) -> ()  [unwired: 1 out]
  n2255 = VISA Close(VISA resource name=w40, error in (no error)=w39) -> (error out=w93:errorcluster)
  n2256 = node-c288(w51) -> ()  [unwired: 1 out]
  n2257 = call <vilib>:"Simple Error Handler.vi"("error in (no error)"=w93) -> ()  [unwired: 1 in, 8 out]
  n2258 = node-c288(w47) -> ()  [unwired: 1 out]
  n2259 = node-c288(w148) -> ()  [unwired: 1 out]
  n2260 = flat-sequence {
    tunnel: w243 -> [w8425]
    tunnel: w245 -> [w8426]
    tunnel: [w8424] -> w224
    tunnel: [w8423] -> w223
    tunnel: w205 -> [_]
    tunnel: w203 -> [_]
    tunnel: w156 -> [_]
    tunnel: w53 -> [_]
    tunnel: w224 -> [w8484]
    tunnel: w223 -> [w8485]
    frame #0 {
      w8422 = FALSE ("AI to FIFO")
      n2261 = xnode "Read/Write Control"("FPGA VI Reference In"=w8426, "error in"=w8425, "AI to FIFO"=w8422, "APD to FIFO"=w8422) -> ("FPGA VI Reference Out"=w8424:T21, "error out"=w8423:errorcluster)
    }
    frame #1 {
      n2262 = xnode "Close FPGA VI Reference"("FPGA VI Reference In"=w8484, "error in"=w8485) -> ("error out"=→"error out":errorcluster)
    }
  }
